vi "A170316-11-Main-large.vi"() -> ()   [LabVIEW 2020]
uses:
  System.Windows.Forms
  Global_Variable/Global.vi
  Database/Global1.vi
  <userlib>/_MGI/Menu Building/MenuTypes/MenuStrip/MGI_MenuStrip.lvclass
  <userlib>/_MGI/Menu Building/MenuItemStatusChange/MGI_MenuItemStatusChange.lvclass
  Libraries/S7/S7.lvlib
panel:
  out "PLC":bool
  out "产品型号":string
  in  "质量报警":bool
  in  "设备缺料":bool
  in  "设备故障":bool
  out "结果字":string
  out "前序状态字":string
  out "前序状态":bool
  in  "菜单":refnum<k24>(container)
  out "检测结果":bool
  in  "批次信息":string[][](table)
  out "提示信息":string
  out "错误":bool
  out "时间字符串":string
  out "日期字符串":string
  out "自动":bool
  out "userStatus":string caption="用户状态"
  out "userName":string caption="用户名"
  out "合格数量":u32
  out "生产数量":u32
  out "追溯码":string
  out "connectionMode":string caption="联机类型"
  in  "更换产品":refnum<vi>
  # "总成检验"
  # "工艺流程"
  # "检测结果："
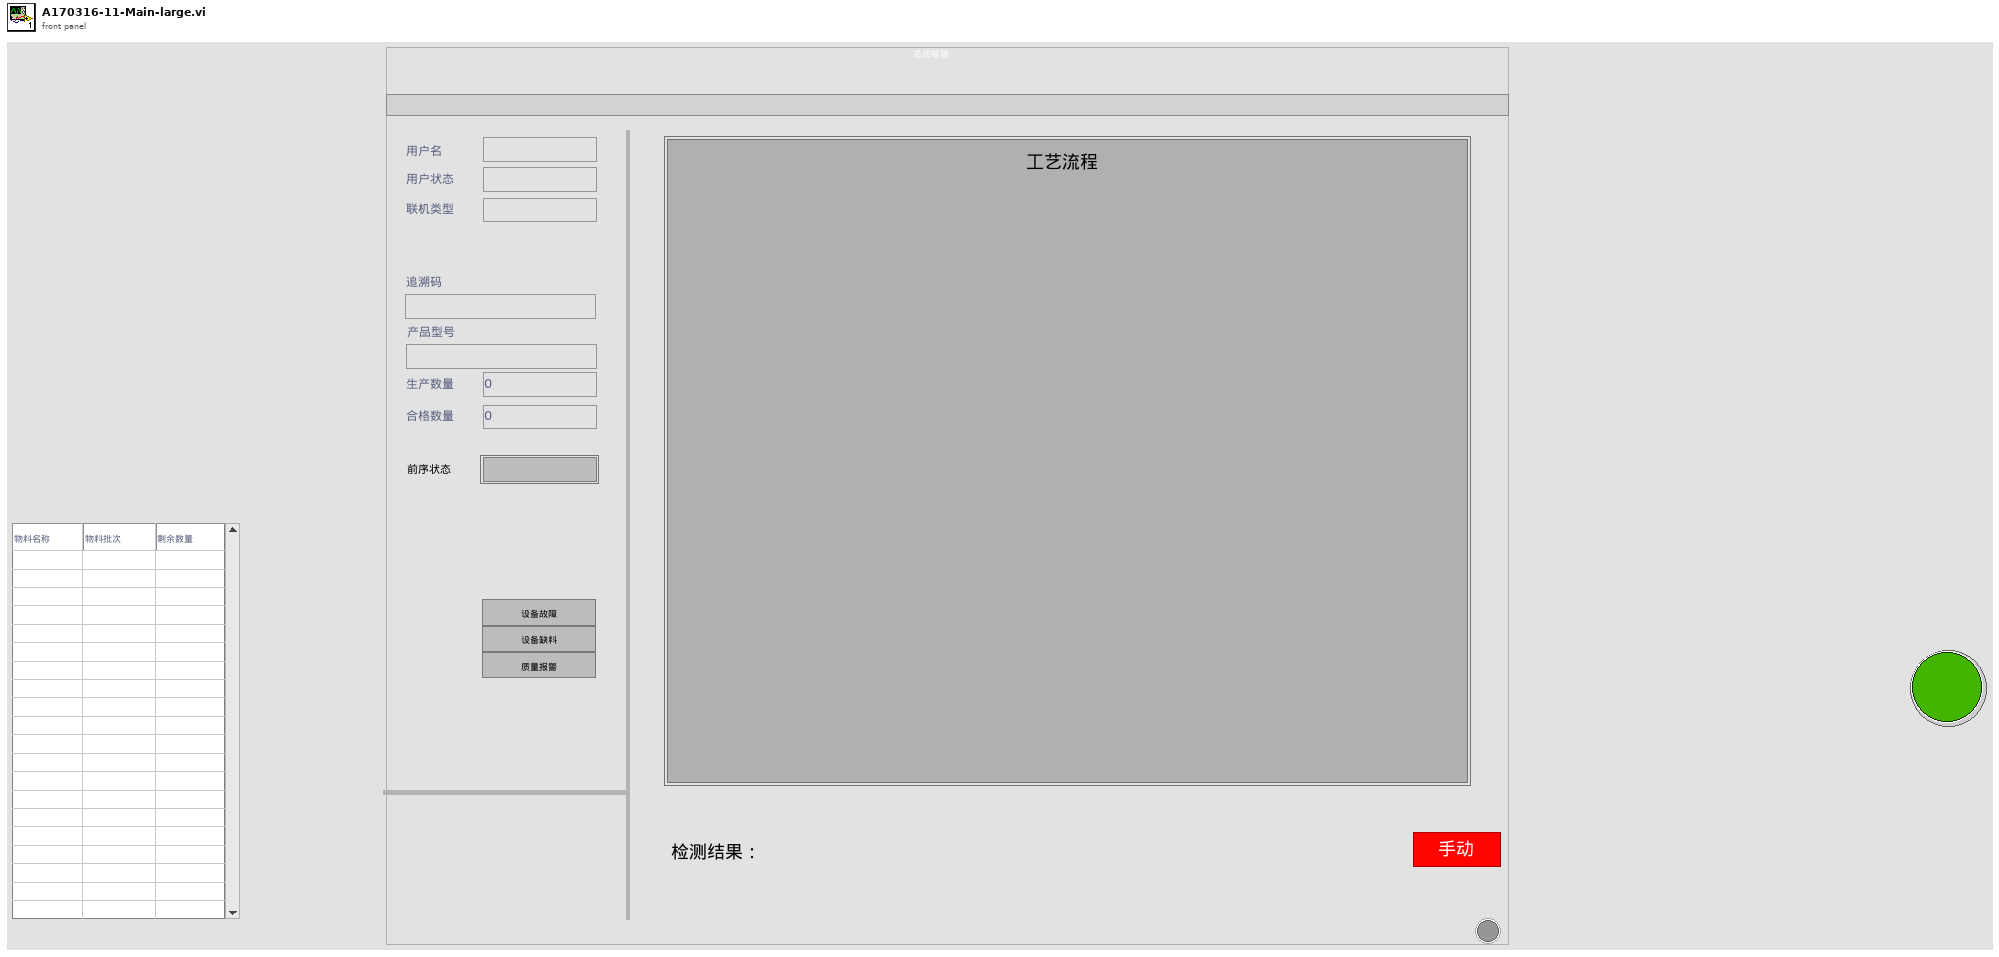
[diagram p1: front panel]
types:
  T1 = typedef "S7.lvlib/Broadcast Events--cluster.ctl" = cluster{"Module Did Init":refnum<user-event>, "Status Updated":refnum<user-event>, "Error Reported":refnum<user-event>, "Module Did Stop":refnum<user-event>, "Update Module Execution Status":refnum<user-event>}
  T2 = enum32{"Invalid", "Standard", "Closed", "Hidden", "Minimized", "Maximized"}
  T3 = enum32{"invalid app kind", "Development System", "Run Time System", "Student Edition", "Embedded LabVIEW", "Evaluation", "Custom"}
  T4 = cluster{"用户编号":string, "用户名":string, "用户密码(密文)":string, "用户权限":string}
  T5 = cluster{"Core":cluster{"Current VI Reference":refnum<vi>, "Close Panel on Exit?":bool}, "Your Boolean data":bool, "Your string data":string}
  T6 = cluster{"Current VI Reference":refnum<vi>, "Close Panel on Exit?":bool}
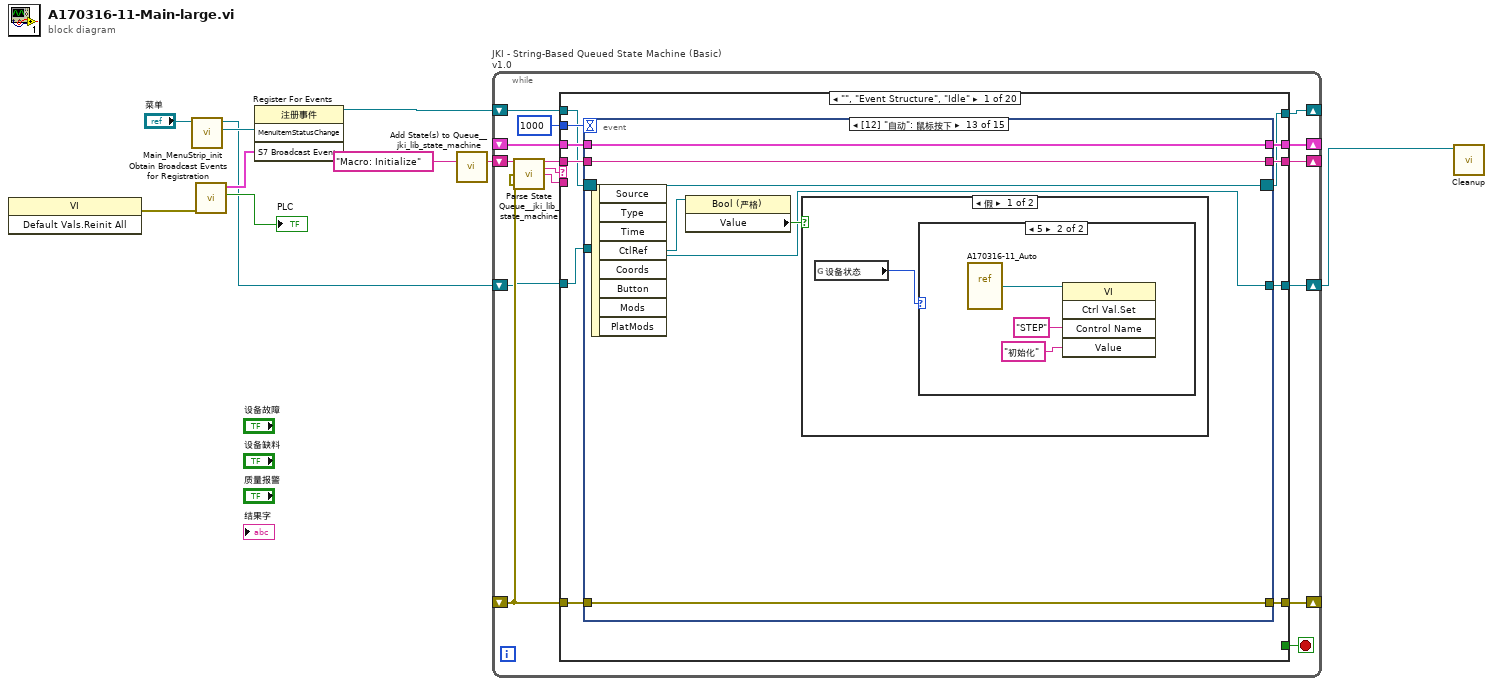
[diagram p0: block diagram]
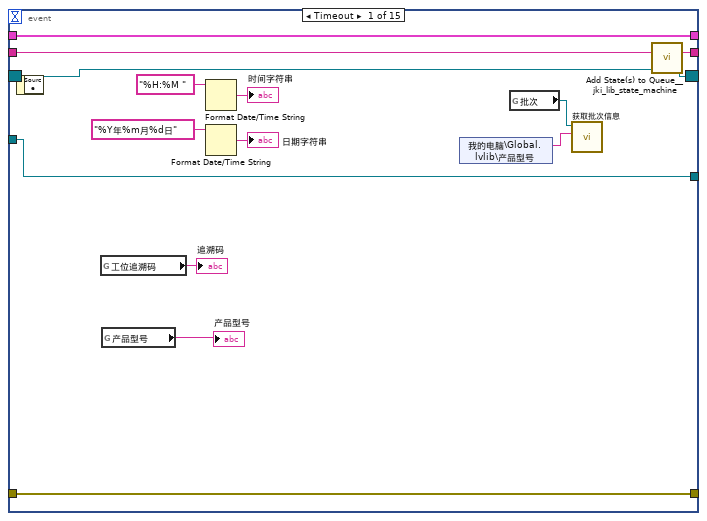
[diagram p2: hidden frame]
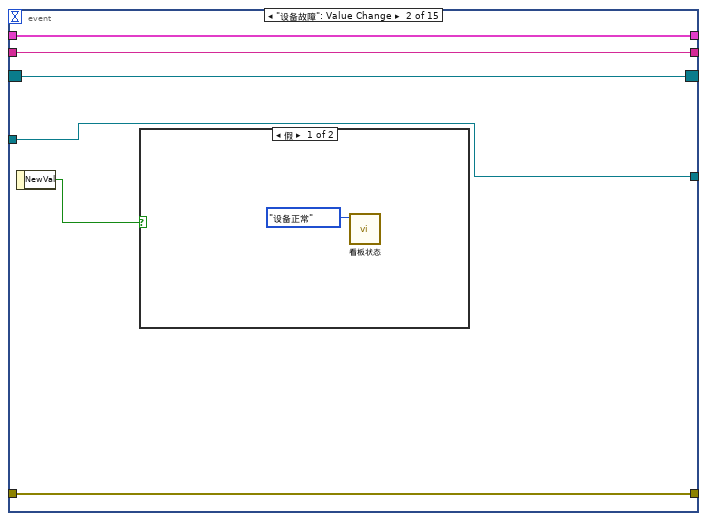
[diagram p3: hidden frame]
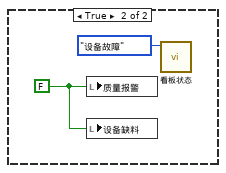
[diagram p4: hidden frame]
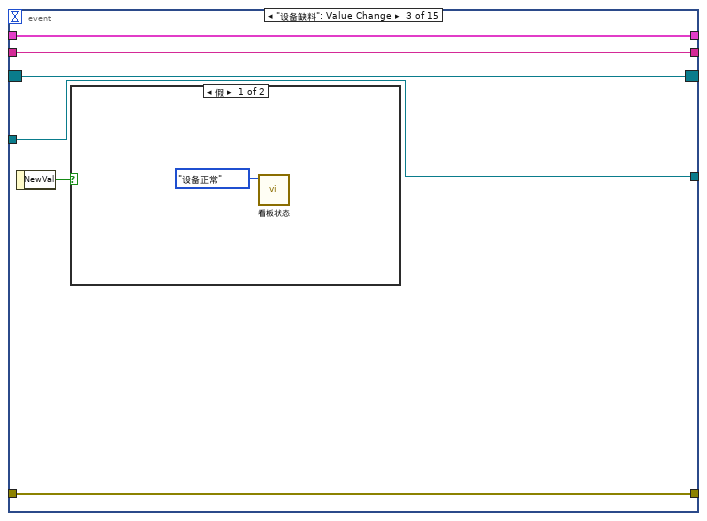
[diagram p5: hidden frame]
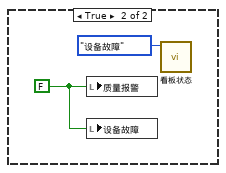
[diagram p6: hidden frame]
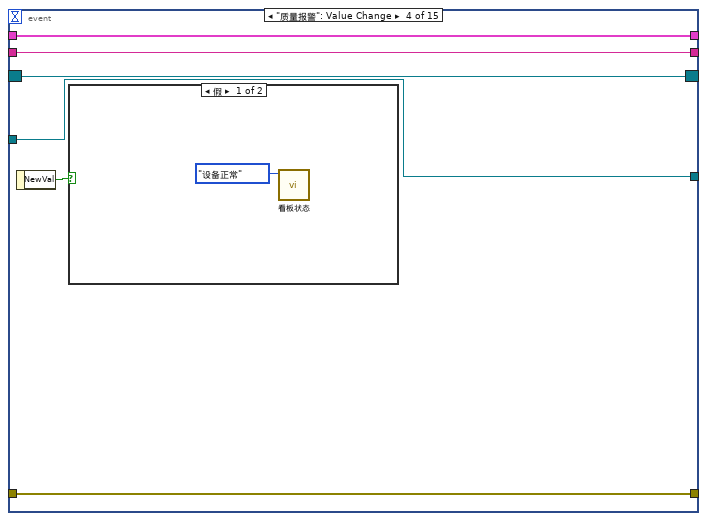
[diagram p7: hidden frame]
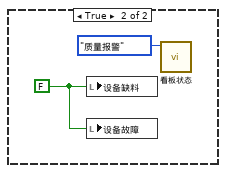
[diagram p8: hidden frame]
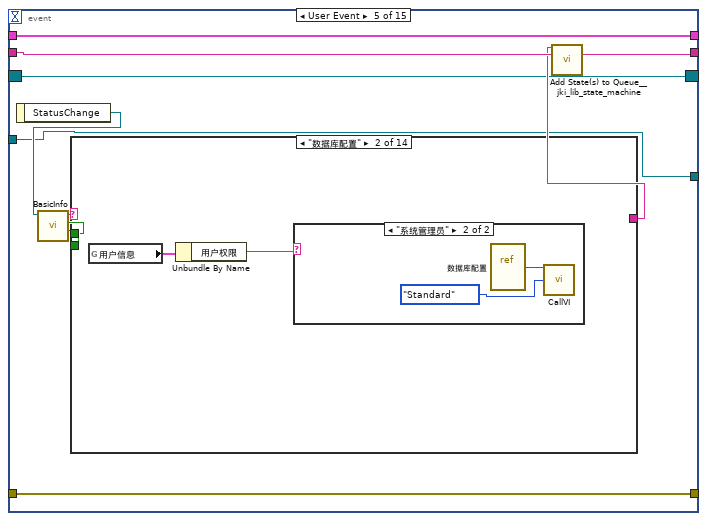
[diagram p9: hidden frame]
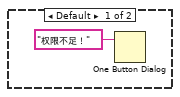
[diagram p11: hidden frame]
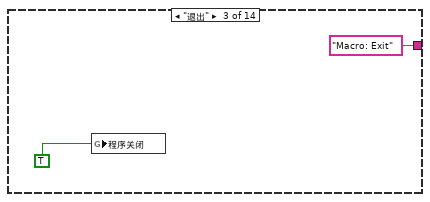
[diagram p12: hidden frame]
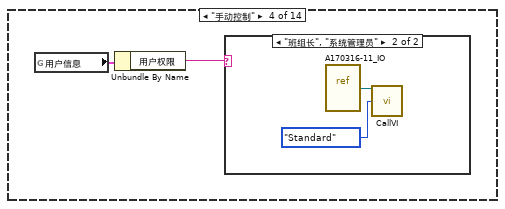
[diagram p13: hidden frame]
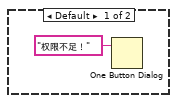
[diagram p14: hidden frame]
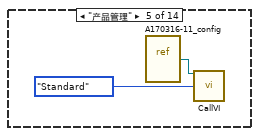
[diagram p15: hidden frame]
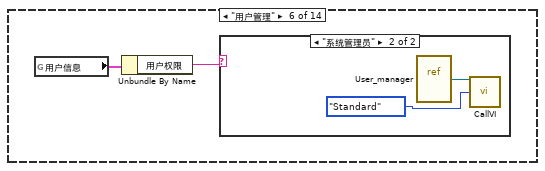
[diagram p16: hidden frame]
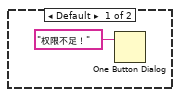
[diagram p17: hidden frame]
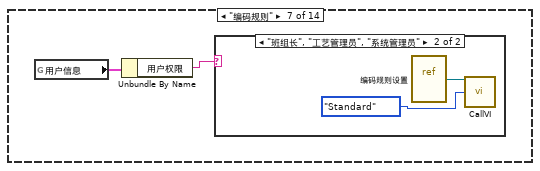
[diagram p18: hidden frame]
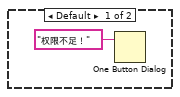
[diagram p19: hidden frame]
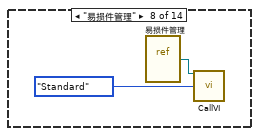
[diagram p20: hidden frame]
diagram:
  n1 = invoke class="VI" method="Default Vals.Reinit All"() -> (error out=w5:errorcluster)  [unwired: 3 in, 2 out]
  n2 = call "Main_MenuStrip_init.vi"("MenuStrip"="菜单") -> ("MenuItemStatusChange"=w7:refnum<user-event>, "Menu out"=w2:refnum<class "MGI_MenuStrip.lvclass">)  [unwired: 9 in]
  n3 = call "Obtain Broadcast Events for Registration.vi"("error in (no error)"=w5) -> ("Already running?"=→"PLC":bool, "S7 Broadcast Events"=w4:T1)  [unwired: 8 in, 1 out]
  n4 = register-events(w7, w4) -> (reference out=w6:refnum<event-registration>)  [unwired: 2 in, 1 out]
  n5 = call <vilib>:"Add State(s) to Queue__jki_lib_state_machine.vi"("State(s) in (\"\")"="Macro: Initialize") -> ("States Out"=w10:string)  [unwired: 14 in]
  n6 = while "JKI - String-Based Queued State Machine (Basic) v1.0" {
    shift-right: [w18] -> _
    shift-left: _ -> [w17]
    shift-right: [w21] -> _
    shift-left: _ -> [w15]
    shift-right: [w20] -> _
    shift-left: w10 -> [w22]
    shift-right: [w12] -> w1
    shift-left: w2 -> [w13]
    shift-right: [w11] -> _
    shift-left: w6 -> [w14]
    stop <- w19 stop-if-true
    n7 = call <vilib>:"Parse State Queue__jki_lib_state_machine.vi"("State Queue"=w22, "Error In (no error)"=w15) -> ("Remaining States"=w24:string, "Current State"=w25:string, "Arguments"=w23:string)  [unwired: 11 in]
    n8 = case shown="\"\", \"Event Structure\", \"Idle\"" w25 {
      selector: w25 -> [_ _ w281 _ _ _ _ _ _ _ _ _ _ _ _ _ _ _ _ _]
      tunnel: w24 -> [w36 w278 w285 w305 w313 w320 w326 w335 w343 w349 w363 w369 w415 w428 w456 w463 w477 w483 w489 w495]
      tunnel: w23 -> [_ _ _ _ _ _ _ _ _ _ _ _ w410 w422 _ _ _ _ _ _]
      tunnel: w17 -> [w34 w275 w283 w296 w310 w318 w323 _ w338 w346 w361 w367 w413 w424 w453 w460 w474 w480 w486 w492]
      tunnel: [w33 w276 w287 w302 errorcluster {"status"=FALSE, "code"=0, "source"=""} ("error out") w317 w324 w332 w339 w347 w358 w366 w411 w425 w454 w461 w475 w481 w487 w493] -> w21
      tunnel: w15 -> [w32 w276 w286 w302 w309 w317 w324 w332 w340 w347 w353 w366 w412 w426 w454 w461 w475 w481 w487 w493]
      tunnel: [w35 w277 w284 w304 w312 w319 w325 w334 w342 w348 w362 w368 w414 w427 w455 w462 w476 w482 w488 w494] -> w20
      tunnel: [_ _ _ _ _ TRUE _ _ _ _ _ _ _ _ _ _ _ _ _ _] -> w19
      tunnel: [w31 w275 w283 w303 w310 w318 w323 w333 w338 w346 w361 w367 w413 w424 w453 w460 w474 w480 w486 w492] -> w18
      tunnel: 1000 ("Timeout") -> [w30 _ _ _ _ _ _ _ _ _ _ _ _ _ _ _ _ _ _ _]
      tunnel: w14 -> [w29 w273 w280 w293 w307 w315 w322 w328 w337 w345 w351 w365 w409 w421 w452 w458 w464 w478 w485 w490]
      tunnel: w13 -> [w28 w274 w279 w292 w306 w314 w321 w327 w336 w344 w350 w364 w408 w420 w451 w457 w465 w479 w484 w491]
      tunnel: [w27 w274 w279 w292 w306 w314 w321 w327 w336 w344 w350 w364 w408 w420 w451 w457 w465 w479 w484 w491] -> w12
      tunnel: [w26 w273 w280 w293 w307 w315 w322 w328 w337 w345 w351 w365 w409 w421 w452 w458 w464 w478 w485 w490] -> w11
      frame "", "Event Structure", "Idle" {
        n9 = event shown="[12] \"自动\": 鼠标按下" {
          selector: w29 -> [w38 w51 w61 w70 w79 w147 w152 w159 w166 w175 w181 w232 w240 w257 w266]
          dyn-events: [w38 w51 w61 w70 w79 w145 w152 w159 w166 w175 w181 w232 w240 w257 w266] -> w26
          timeout: w30 -> [_ _ _ _ _ _ _ _ _ _ _ _ _ _ _]
          tunnel: w36 -> [w50 w54 w63 w72 w83 w137 w154 w161 w168 w177 w184 w236 w244 w264 w269]
          tunnel: [w49 w54 w63 w72 w82 w137 w153 w160 w167 w176 w182 w237 w244 w263 w270] -> w35
          tunnel: w34 -> [w47 w55 w64 w73 w84 w138 w155 w162 w169 w178 w183 w238 w245 w261 w272]
          tunnel: [w48 w53 w62 w71 w80 w139 w150 w157 w165 w171 w185 w235 w243 w262 w271] -> w33
          tunnel: w32 -> [w48 w53 w62 w71 w80 w149 w150 w157 w165 w172 w185 w235 w243 w262 w271]
          tunnel: [w47 w55 w64 w73 w84 w138 w155 w162 w169 w178 w183 w238 w245 w261 w272] -> w31
          tunnel: w28 -> [w37 w52 w60 w69 w78 w136 w156 w163 w170 w179 w180 w231 w239 w256 w265]
          tunnel: [w37 w52 w60 w69 w78 w136 w156 w163 w170 w179 w180 w231 w239 w256 w265] -> w27
          event Timeout {
            n10 = event-data() -> ()  [unwired: 1 in, 1 out]
            n11 = global read "Global1.vi" "工位追溯码"() -> (→"追溯码":string)
            n12 = global read "Global.vi" "产品型号"() -> (→"产品型号":string)
            n13 = Format Date/Time String(time format string (%c)="%H:%M ") -> (date/time string=→"时间字符串":string)  [unwired: 2 in]
            n14 = Format Date/Time String(time format string (%c)="%Y年%m月%d日") -> (date/time string=→"日期字符串":string)  [unwired: 2 in]
            n15 = shared-variable "我的电脑\\Global.lvlib\\产品型号"() -> (w42:string)  [unwired: 1 in, 1 out]
            n16 = global read "Global.vi" "批次"() -> (w41:refnum<vi>)
            n17 = call "获取批次信息.vi"("产品型号"=w42, "Tbl引用句柄"=w41) -> ()  [unwired: 8 in, 2 out]
            n18 = call <vilib>:"Add State(s) to Queue__jki_lib_state_machine.vi"("State(s) in (\"\")"=w50) -> ("States Out"=w49:string)  [unwired: 14 in]
          }
          event "设备故障": Value Change {
            n19 = event-data() -> ("NewVal"=w56:bool)  [unwired: 1 in]
            n20 = case shown="假" w56 {
              frame False {
                n21 = call "看板状态.vi"("设备状态"=enum16{"设备离线", "设备正常", "设备缺料", "设备故障", "质量报警"}."设备正常") -> ()  [unwired: 10 in, 1 out]
              }
              frame True {
                w58 = FALSE ("质量报警")
                n22 = local write "质量报警"(w58) -> ()
                n23 = local write "设备缺料"(w58) -> ()
                n24 = call "看板状态.vi"("设备状态"=enum16{"设备离线", "设备正常", "设备缺料", "设备故障", "质量报警"}."设备故障") -> ()  [unwired: 10 in, 1 out]
              }
            }
          }
          event "设备缺料": Value Change {
            n25 = event-data() -> ("NewVal"=w65:bool)  [unwired: 1 in]
            n26 = case shown="假" w65 {
              frame False {
                n27 = call "看板状态.vi"("设备状态"=enum16{"设备离线", "设备正常", "设备缺料", "设备故障", "质量报警"}."设备正常") -> ()  [unwired: 10 in, 1 out]
              }
              frame True {
                w67 = FALSE ("质量报警")
                n28 = local write "质量报警"(w67) -> ()
                n29 = local write "设备故障"(w67) -> ()
                n30 = call "看板状态.vi"("设备状态"=enum16{"设备离线", "设备正常", "设备缺料", "设备故障", "质量报警"}."设备故障") -> ()  [unwired: 10 in, 1 out]
              }
            }
          }
          event "质量报警": Value Change {
            n31 = event-data() -> ("NewVal"=w74:bool)  [unwired: 1 in]
            n32 = case shown="假" w74 {
              frame False {
                n33 = call "看板状态.vi"("设备状态"=enum16{"设备离线", "设备正常", "设备缺料", "设备故障", "质量报警"}."设备正常") -> ()  [unwired: 10 in, 1 out]
              }
              frame True {
                w76 = FALSE ("质量报警")
                n34 = local write "设备缺料"(w76) -> ()
                n35 = local write "设备故障"(w76) -> ()
                n36 = call "看板状态.vi"("设备状态"=enum16{"设备离线", "设备正常", "设备缺料", "设备故障", "质量报警"}."质量报警") -> ()  [unwired: 10 in, 1 out]
              }
            }
          }
          event User Event {
            n37 = event-data() -> ("StatusChange"=w85:refnum<class "MGI_MenuItemStatusChange.lvclass">)  [unwired: 1 in]
            n38 = call <userlib>:"BasicInfo.vi"("MGI_MenuItemStatusChange in"=w85) -> ("Enabled?"=w88:bool, "Checked?"=w87:bool, "Tag"=w86:string)  [unwired: 7 in, 1 out]
            n39 = case shown="\"数据库配置\"" w86 {
              tunnel: w87 -> [_ _ _ _ _ _ _ _ _ _ _ _ _ _]
              tunnel: w88 -> [_ _ _ _ _ _ _ _ _ _ _ _ _ _]
              tunnel: [_ _ "Macro: Exit" _ _ _ _ _ _ _ _ _ _ _] -> w81
              frame Default {
              }
              frame "数据库配置" {
                n40 = global read "Global1.vi" "用户信息"() -> (w89:T4)
                n41 = Unbundle By Name(w89) -> ("用户权限"=w90:string)
                n42 = case shown="\"系统管理员\"" w90 {
                  frame Default {
                    n43 = One Button Dialog(message="权限不足！" ("消息")) -> ()  [unwired: 1 in, 1 out]
                  }
                  frame "系统管理员" {
                    n44 = vi-ref "数据库配置.vi"() -> (w93:refnum<vi>)
                    n45 = call "CallVI.vi"("VI引用"=w93, "状态"=T2."Standard") -> ()  [unwired: 11 in, 3 out]
                  }
                }
              }
              frame "退出" {
                n46 = global write "Global.vi" "程序关闭"(TRUE ("程序关闭")) -> ()
              }
              frame "手动控制" {
                n47 = global read "Global1.vi" "用户信息"() -> (w97:T4)
                n48 = Unbundle By Name(w97) -> ("用户权限"=w96:string)
                n49 = case shown="\"班组长\", \"系统管理员\"" w96 {
                  frame Default {
                    n50 = One Button Dialog(message="权限不足！" ("消息")) -> ()  [unwired: 1 in, 1 out]
                  }
                  frame "班组长", "系统管理员" {
                    n51 = vi-ref "A170316-11_IO.vi"() -> (w100:refnum<vi>)
                    n52 = call "CallVI.vi"("VI引用"=w100, "状态"=T2."Standard") -> ()  [unwired: 11 in, 3 out]
                  }
                }
              }
              frame "产品管理" {
                n53 = vi-ref "A170316-11_config.vi"() -> (w102:refnum<vi>)
                n54 = call "CallVI.vi"("VI引用"=w102, "状态"=T2."Standard") -> ()  [unwired: 11 in, 3 out]
              }
              frame "用户管理" {
                n55 = global read "Global1.vi" "用户信息"() -> (w104:T4)
                n56 = Unbundle By Name(w104) -> ("用户权限"=w103:string)
                n57 = case shown="\"系统管理员\"" w103 {
                  frame Default {
                    n58 = One Button Dialog(message="权限不足！" ("消息")) -> ()  [unwired: 1 in, 1 out]
                  }
                  frame "系统管理员" {
                    n59 = vi-ref "User_manager.vi"() -> (w107:refnum<vi>)
                    n60 = call "CallVI.vi"("VI引用"=w107, "状态"=T2."Standard") -> ()  [unwired: 11 in, 3 out]
                  }
                }
              }
              frame "编码规则" {
                n61 = global read "Global1.vi" "用户信息"() -> (w109:T4)
                n62 = Unbundle By Name(w109) -> ("用户权限"=w108:string)
                n63 = case shown="\"班组长\", \"工艺管理员\", \"系统管理员\"" w108 {
                  frame Default {
                    n64 = One Button Dialog(message="权限不足！" ("消息")) -> ()  [unwired: 1 in, 1 out]
                  }
                  frame "班组长", "工艺管理员", "系统管理员" {
                    n65 = vi-ref "编码规则设置.vi"() -> (w112:refnum<vi>)
                    n66 = call "CallVI.vi"("VI引用"=w112, "状态"=T2."Standard") -> ()  [unwired: 11 in, 3 out]
                  }
                }
              }
              frame "易损件管理" {
                n67 = vi-ref "易损件管理.vi"() -> (w114:refnum<vi>)
                n68 = call "CallVI.vi"("VI引用"=w114, "状态"=T2."Standard") -> ()  [unwired: 11 in, 3 out]
              }
              frame "物料批次管理" {
                n69 = vi-ref "批次管理.vi"() -> (w116:refnum<vi>)
                n70 = call "CallVI.vi"("VI引用"=w116, "状态"=T2."Standard") -> ()  [unwired: 11 in, 3 out]
              }
              frame "报表" {
                n71 = call "文件对话框2"("start path"=path "D:/report", "prompt"="打开报表", "pattern (all files)"="*.doc;*.docx", "pattern label"="Word 文档") -> ("selected path"=w117:path, "error out"=w118:errorcluster)  [unwired: 8 in, 2 out]
                n72 = case shown="无错误" w118 {
                  selector: w118 -> [w124 w126]
                  tunnel: w117 -> [w125 _]
                  frame No Error {
                    w123 = 1 items=["Normal", "Maximize", "Minimize"] ("cpubbs_WindowState")
                    n73 = call "Open_Word.vi"("File Path"=w125, "cpubbs_WindowState"=w123, "错误输入（无错误）"=w124) -> ()  [unwired: 12 in, 1 out]
                  }
                  frame Error {
                    n74 = call <vilib>:"Clear Errors.vi"("error in (no error)"=w126) -> ()  [unwired: 5 in, 2 out]
                  }
                }
              }
              frame "报警信息" {
                n75 = vi-ref "报警信息.vi"() -> (w128:refnum<vi>)
                n76 = call "CallVI.vi"("VI引用"=w128, "状态"=T2."Standard") -> ()  [unwired: 11 in, 3 out]
              }
              frame "关于" {
                n77 = vi-ref "About.vi"() -> (w130:refnum<vi>)
                n78 = call "CallVI.vi"("VI引用"=w130, "状态"=T2."Standard") -> ()  [unwired: 11 in, 3 out]
              }
              frame "设备管理" {
                n79 = vi-ref "注册设备.vi"() -> (w132:refnum<vi>)
                n80 = call "CallVI.vi"("VI引用"=w132, "状态"=T2."Standard") -> ()  [unwired: 11 in, 3 out]
              }
              frame "操作演示" {
                n81 = call <vilib>:"Application Directory.vi"() -> ("Application Directory"=w135:path)
                n82 = Build Path(base path=w135, name or relative path="操作演示" ("名称或相对路径")) -> (appended path=w134:path)
                n83 = call "自动播放ppt.vi"("路径"=w134) -> ()  [unwired: 10 in, 1 out]
              }
            }
            n84 = call <vilib>:"Add State(s) to Queue__jki_lib_state_machine.vi"("State(s) in Front (\"\")"=w81, "State(s) in (\"\")"=w83) -> ("States Out"=w82:string)  [unwired: 13 in]
          }
          event "PLC": Value Change; "PLC": Mouse Down {
            n85 = event-data() -> ()  [unwired: 1 in, 4 out]
            n86 = call "Start Module.vi"("error in (no error)"=w149) -> ("Wait for Event Sync?"=w143:bool, "S7 Broadcast Events"=w146:T1, "Module Was Already Running?"=w148:bool)  [unwired: 7 in, 1 out]
            n87 = local write "PLC"(w148) -> ()
            n88 = register-events(reference=w147, w146) -> (reference out=w145:refnum<event-registration>, error out=w144:errorcluster)  [unwired: 2 in]
            n89 = call "Synchronize Module Events.vi"("error in (no error)"=w144, "Wait for Event Sync?"=w143) -> ("error out"=w142:errorcluster)  [unwired: 9 in]
            n90 = call "Init S7 Link.vi"("error in (no error)"=w142, "超时"=1000, "IP"="192.168.0.91") -> ("error out"=w139:errorcluster)  [unwired: 8 in]
          }
          event User Event {
            n91 = event-data() -> ("Init?"=w151:bool)  [unwired: 1 in, 1 out]
            n92 = local write "PLC"(w151) -> ()
            n93 = call <vilib>:"Add State(s) to Queue__jki_lib_state_machine.vi"("State(s) in (\"\")"=w154) -> ("States Out"=w153:string)  [unwired: 14 in]
          }
          event User Event {
            n94 = event-data() -> ("Running?"=w158:bool)  [unwired: 1 in]
            n95 = local write "PLC"(w158) -> ()
            n96 = call <vilib>:"Add State(s) to Queue__jki_lib_state_machine.vi"("State(s) in (\"\")"=w161) -> ("States Out"=w160:string)  [unwired: 14 in]
          }
          event User Event {
            n97 = event-data() -> ()  [unwired: 1 in, 3 out]
            n98 = local write "PLC"(FALSE ("PLC")) -> ()
            n99 = call <vilib>:"Add State(s) to Queue__jki_lib_state_machine.vi"("State(s) in (\"\")"=w168) -> ("States Out"=w167:string)  [unwired: 14 in]
          }
          event User Event {
            n100 = event-data() -> ("Error"=w173:errorcluster)  [unwired: 1 in, 2 out]
            n101 = Merge Errors(w173, w172) -> (w171:errorcluster)
            n102 = call <vilib>:"Add State(s) to Queue__jki_lib_state_machine.vi"("State(s) in Front (\"\")"="S7: Initialize\nIdle" ("State(s) in Front (\"\")"), "State(s) in (\"\")"=w177) -> ("States Out"=w176:string)  [unwired: 13 in]
          }
          event Menu Selection (User) {
            n103 = event-data() -> ("ItemTag"=w186:string)  [unwired: 1 in, 6 out]
            n104 = case shown="\"退出\"" w186 {
              frame "假", Default {
              }
              frame "数据库配置" {
                n105 = shared-variable "我的电脑\\Global.lvlib\\操作者权限"() -> (w187:string)  [unwired: 1 in, 1 out]
                n106 = case shown="\"系统管理员\"" w187 {
                  frame Default {
                    n107 = One Button Dialog(message="权限不足！" ("消息")) -> ()  [unwired: 1 in, 1 out]
                  }
                  frame "系统管理员" {
                    n108 = vi-ref "数据库配置.vi"() -> (w190:refnum<vi>)
                    n109 = call "CallVI.vi"("VI引用"=w190, "状态"=T2."Standard") -> ()  [unwired: 11 in, 3 out]
                  }
                }
              }
              frame "退出" {
                n110 = Quit LabVIEW() -> ()  [unwired: 1 in]
              }
              frame "手动控制" {
                n111 = shared-variable "我的电脑\\Global.lvlib\\操作者权限"() -> (w191:string)  [unwired: 1 in, 1 out]
                n112 = case shown="\"班组长\", \"系统管理员\"" w191 {
                  frame Default {
                    n113 = One Button Dialog(message="权限不足！" ("消息")) -> ()  [unwired: 1 in, 1 out]
                  }
                  frame "班组长", "系统管理员" {
                    n114 = vi-ref "A170316-11_IO.vi"() -> (w194:refnum<vi>)
                    n115 = call "CallVI.vi"("VI引用"=w194, "状态"=T2."Standard") -> ()  [unwired: 11 in, 3 out]
                  }
                }
              }
              frame "半自动控制" {
                n116 = disable-structure shown="禁用" {
                  frame Disabled {
                    n117 = shared-variable "我的电脑\\Global.lvlib\\操作者权限"() -> (w195:string)  [unwired: 1 in, 1 out]
                    n118 = case shown="\"班组长\", \"系统管理员\"" w195 {
                      frame Default {
                        n119 = One Button Dialog(message="权限不足！" ("消息")) -> ()  [unwired: 1 in, 1 out]
                      }
                      frame "班组长", "系统管理员" {
                        n120 = call "CallVI.vi"("VI引用"=refnum<vi> refnum, "状态"=T2."Maximized") -> ()  [unwired: 11 in, 3 out]
                      }
                    }
                  }
                  frame Enabled {
                    n121 = One Button Dialog(message="当前设备不具备半自动功能！" ("消息")) -> ()  [unwired: 1 in, 1 out]
                  }
                }
              }
              frame "产品管理" {
                n122 = vi-ref "A170316-11_config.vi"() -> (w201:refnum<vi>)
                n123 = call "CallVI.vi"("VI引用"=w201, "状态"=T2."Standard") -> ()  [unwired: 11 in, 3 out]
              }
              frame "系统配置" {
              }
              frame "用户管理" {
                n124 = shared-variable "我的电脑\\Global.lvlib\\操作者权限"() -> (w202:string)  [unwired: 1 in, 1 out]
                n125 = case shown="\"系统管理员\"" w202 {
                  frame Default {
                    n126 = One Button Dialog(message="权限不足！" ("消息")) -> ()  [unwired: 1 in, 1 out]
                  }
                  frame "系统管理员" {
                    n127 = vi-ref "User_manager.vi"() -> (w205:refnum<vi>)
                    n128 = call "CallVI.vi"("VI引用"=w205, "状态"=T2."Standard") -> ()  [unwired: 11 in, 3 out]
                  }
                }
              }
              frame "编码规则" {
                n129 = shared-variable "我的电脑\\Global.lvlib\\操作者权限"() -> (w206:string)  [unwired: 1 in, 1 out]
                n130 = case shown="\"班组长\", \"工艺管理员\", \"系统管理员\"" w206 {
                  frame Default {
                    n131 = One Button Dialog(message="权限不足！" ("消息")) -> ()  [unwired: 1 in, 1 out]
                  }
                  frame "班组长", "工艺管理员", "系统管理员" {
                    n132 = vi-ref "编码规则设置.vi"() -> (w209:refnum<vi>)
                    n133 = call "CallVI.vi"("VI引用"=w209, "状态"=T2."Standard") -> ()  [unwired: 11 in, 3 out]
                  }
                }
              }
              frame "易损件管理" {
                n134 = vi-ref "易损件管理.vi"() -> (w211:refnum<vi>)
                n135 = call "CallVI.vi"("VI引用"=w211, "状态"=T2."Standard") -> ()  [unwired: 11 in, 3 out]
              }
              frame "物料批次管理" {
                n136 = vi-ref "批次管理.vi"() -> (w213:refnum<vi>)
                n137 = call "CallVI.vi"("VI引用"=w213, "状态"=T2."Standard") -> ()  [unwired: 11 in, 3 out]
              }
              frame "打开报表" {
                n138 = call "文件对话框"("start path"=path "D:/report", "prompt"="打开报表", "pattern (all files)"="*.doc;*.docx", "pattern label"="Word 文档") -> ("selected path"=w214:path, "error out"=w215:errorcluster)  [unwired: 8 in, 2 out]
                n139 = case shown="无错误" w215 {
                  selector: w215 -> [w221 w223]
                  tunnel: w214 -> [w222 _]
                  frame No Error {
                    w220 = 1 items=["Normal", "Maximize", "Minimize"] ("cpubbs_WindowState")
                    n140 = call "Open_Word.vi"("File Path"=w222, "cpubbs_WindowState"=w220, "错误输入（无错误）"=w221) -> ()  [unwired: 12 in, 1 out]
                  }
                  frame Error {
                    n141 = call <vilib>:"Clear Errors.vi"("error in (no error)"=w223) -> ()  [unwired: 5 in, 2 out]
                  }
                }
              }
              frame "报警信息" {
                n142 = vi-ref "报警信息.vi"() -> (w225:refnum<vi>)
                n143 = call "CallVI.vi"("VI引用"=w225, "状态"=T2."Standard") -> ()  [unwired: 11 in, 3 out]
              }
              frame "关于" {
                n144 = vi-ref "About.vi"() -> (w227:refnum<vi>)
                n145 = call "CallVI.vi"("VI引用"=w227, "状态"=T2."Standard") -> ()  [unwired: 11 in, 3 out]
              }
              frame "操作演示" {
                n146 = call <vilib>:"Application Directory.vi"() -> ("Application Directory"=w230:path)
                n147 = Build Path(base path=w230, name or relative path="操作演示" ("名称或相对路径")) -> (appended path=w229:path)
                n148 = call "自动播放ppt.vi"("路径"=w229) -> ()  [unwired: 10 in, 1 out]
              }
            }
            n149 = call <vilib>:"Add State(s) to Queue__jki_lib_state_machine.vi"("State(s) in (\"\")"=w184) -> ("States Out"=w182:string)  [unwired: 14 in]
          }
          event "错误": Mouse Down {
            n150 = event-data() -> ()  [unwired: 1 in, 8 out]
            n151 = vi-ref "报警信息.vi"() -> (w234:refnum<vi>)
            n152 = call "CallVI.vi"("VI引用"=w234, "状态"=T2."Standard") -> ()  [unwired: 11 in, 3 out]
            n153 = call <vilib>:"Add State(s) to Queue__jki_lib_state_machine.vi"("State(s) in (\"\")"=w236) -> ("States Out"=w237:string)  [unwired: 14 in]
          }
          event "自动": Mouse Down {
            n154 = event-data() -> ("CtlRef"=w242:refnum<vi>)  [unwired: 1 in, 7 out]
            n155 = property class="Bool (严格)"(reference=w242) -> ("Value"=w241:bool)  [unwired: 1 in, 2 out]
            n156 = case shown="假" w241 {
              frame False {
                n157 = global read "Global.vi" "设备状态"() -> (w246:i32)
                n158 = case shown="5" w246 {
                  frame 0, Default {
                    n159 = call "浮动通知.vi"("通知内容"="请复位！") -> ()  [unwired: 11 in]
                  }
                  frame 5 {
                    n160 = vi-ref "A170316-11_Auto.vi"() -> (w250:refnum<vi>)
                    n161 = invoke class="VI" method="Ctrl Val.Set"(reference=w250, "Control Name"="STEP" ("控件名"), "Value"="初始化" ("控件名")) -> ()  [unwired: 2 in, 5 out]
                  }
                }
              }
              frame True {
                n162 = Two Button Dialog(message="自动程序运行中，\n是否切换为手动？" ("消息")) -> (T button?=w251:bool)  [unwired: 2 in]
                n163 = case shown="真" w251 {
                  frame False {
                  }
                  frame True {
                    n164 = vi-ref "A170316-11_Auto.vi"() -> (w255:refnum<vi>)
                    n165 = invoke class="VI" method="Ctrl Val.Set"(reference=w255, "Control Name"="STEP" ("控件名"), "Value"="手动" ("控件名")) -> ()  [unwired: 2 in, 5 out]
                  }
                }
              }
            }
          }
          event Panel Close? {
            n166 = event-data() -> ()  [unwired: 1 in, 1 out]
            n167 = global write "Global.vi" "程序关闭"(TRUE ("程序关闭")) -> ()
            n168 = event-data("Discard?"=TRUE) -> ()  [unwired: 1 in, 1 out]
            n169 = call <vilib>:"Add State(s) to Queue__jki_lib_state_machine.vi"("State(s) in Front (\"\")"="Macro: Exit", "State(s) in (\"\")"=w264) -> ("States Out"=w263:string)  [unwired: 13 in]
          }
          event "更换产品": Value Change {
            n170 = event-data() -> ("NewVal"=w268:refnum<vi>)  [unwired: 1 in, 5 out]
            n171 = control-ref of="子面板"() -> (w267:refnum<vi>)
            n172 = call "Call_SubPanal.vi"("VI引用句柄"=w268, "SubPnl引用句柄"=w267) -> ()  [unwired: 9 in, 1 out]
            n173 = call <vilib>:"Add State(s) to Queue__jki_lib_state_machine.vi"("State(s) in (\"\")"=w269) -> ("States Out"=w270:string)  [unwired: 14 in]
          }
        }
      }
      frame "---------- Core ----------" {
        n174 = call <vilib>:"Add State(s) to Queue__jki_lib_state_machine.vi"("State(s) in (\"\")"=w278) -> ("States Out"=w277:string)  [unwired: 14 in]
      }
      frame Default {
        w290 = 42 items=["No error", "Argument error", "Memory is full", "Out of zone", "End of file", "File already open", "Generic file I/O error", "File not found", "File permission error", "Disk is full", "Duplicate path", "Too many files open", "System feature not enabled", "Resource file not found", "Cannot add resource", "Resource not found", "Image not found", "Image memory error", "Pen does not exist", "Config type invalid", "Config token not found", "Config parse error", "Config memory error", "Bad external code format", "Bad external code offset", "External code not present", "Null window", "Destroy window error", "Null menu", "Print aborted", "Bad print record", "Print driver error", "Windows error during printing", "Memory error during printing", "Print dialog error", "Generic print error", "Invalid device refnum", "Device not found", "Device parameter error", "Device unit error", "Cannot open device", "Device call aborted", "Generic error", "Cancelled by user", "Object ID too low", "Object ID too high", "Object not in heap", "Unknown heap", "Unknown object (invalid DefProc)", "Unknown object (DefProc not in table)", "Message out of range", "Invalid (null) method", "Unknown message", "Manager call not supported", "Bad address", "Network operation in progress", "Network operation timed out", "Connection is busy", "Network attribute not supported", "Network error", "Address in use", "System out of memory", "Connection aborted", "Connection refused", "Not connected", "Already connected", "Connection closed", "Initialization error (interapplication manager)", "Bad occurrence", "Wait on unbound occurrence handler", "Occurrence queue overflow", "Datalog type conflict", "Unused", "Unrecognized type (interapplication manager)", "Memory corrupt", "Failed to make temporary DLL", "Old CIN version", "Drag socket not found", "Failed to load drop-object", "Failed to register OLE object", "Failed to release OLE object", "Format specifier type mismatch", "Unknown format specifier", "Too few format specifiers", "Too many format specifiers", "Scan failed", "Newer CIN version", "Error converting to variant", "Runtime menu error", "Password tampered", "Variant attribute not found", "Incompatible variant data type", "Event data is not available", "Event Store is not present", "Occurrence is not found", "Event Queue is not created", "Event info is not available", "Refnum passed is NULL", "Error retrieving Class GUID", "Error retrieving CoClass GUID", "Error retrieving TypeLib GUID.", "Bad built application magic bytes.", "Specific driver is different from the specific driver associated with the Logical Name.", "There is no session opened to the class driver.", "Max Error", "MAX - Error with config objects", "MAX - Error loading configuration", "MAX - Group not supported"]
        # "Current State"
        n175 = Format Into String(format string="Software Exception: Unhandled State \"%s\"." ("message"), error in=w286, w281) -> (resulting string=w289:string, error out=w288:errorcluster)  [unwired: 1 in]
        n176 = call <vilib>:"Error Cluster From Error Code.vi"("show call chain? (False)"=TRUE, "error in (no error)"=w288, "error message (\"\")"=w289, "error code (0)"=w290) -> ("error out"=w287:errorcluster)  [unwired: 5 in]
        n177 = call <vilib>:"Add State(s) to Queue__jki_lib_state_machine.vi"("State(s) in (\"\")"=w285) -> ("States Out"=w284:string)  [unwired: 14 in]
      }
      frame "Initialize Core Data" {
        # "originally closed?"
        # "exe?"
        n178 = property class="VI"() -> ("Front Panel.Open"=w301:bool)  [unwired: 2 in, 2 out]
        n179 = property class="App"() -> ("App.Kind"=w300:T3)  [unwired: 2 in, 2 out]
        n180 = control-ref of="Current VI Reference"() -> (w294:refnum<vi>)
        n181 = Not(x=w301) -> (.not. x?=w298:bool)
        n182 = Equal?(x=w300, y=T3."Run Time System" ("Application:Kind")) -> (x = y?=w297:bool)
        n183 = Or(x=w298, y=w297) -> (x .or. y?=w295:bool)
        n184 = Bundle By Name(cluster=w296, "Core.Current VI Reference"=w294, "Core.Close Panel on Exit?"=w295) -> (w303:T5)
        n185 = call <vilib>:"Add State(s) to Queue__jki_lib_state_machine.vi"("State(s) in (\"\")"=w305) -> ("States Out"=w304:string)  [unwired: 14 in]
      }
      frame "Error Handler" {
        n186 = call <vilib>:"General Error Handler.vi"("error in (no error)"=w309) -> ()  [unwired: 10 in, 5 out]
        n187 = call <vilib>:"Add State(s) to Queue__jki_lib_state_machine.vi"("State(s) in Front (\"\")"="/* Post Error States", "State(s) in (\"\")"=w313) -> ("States Out"=w312:string)  [unwired: 13 in]
      }
      frame "Exit" {
        n188 = call <vilib>:"Add State(s) to Queue__jki_lib_state_machine.vi"("State(s) in (\"\")"=w320) -> ("States Out"=w319:string)  [unwired: 14 in]
      }
      frame "---------- Data ----------" {
        n189 = call <vilib>:"Add State(s) to Queue__jki_lib_state_machine.vi"("State(s) in (\"\")"=w326) -> ("States Out"=w325:string)  [unwired: 14 in]
      }
      frame "Data: Initialize" {
        w329 = T6 {"Current VI Reference"=refnum, "Close Panel on Exit?"=FALSE}  # Core
        w331 = TRUE  # Your Boolean data
        w330 = ""  # Your string data
        n190 = Bundle("Core"=w329, "Your Boolean data"=w331, "Your string data"=w330) -> (w333:T5)  [unwired: 1 in]
        n191 = call <vilib>:"Add State(s) to Queue__jki_lib_state_machine.vi"("State(s) in (\"\")"=w335) -> ("States Out"=w334:string)  [unwired: 14 in]
      }
      frame "Data: Cleanup" {
        n192 = Unbundle By Name(w338) -> ("Core.Current VI Reference"=w341:refnum<vi>)
        n193 = Close Reference(reference=w341, error in (no error)=w340) -> (error out=w339:errorcluster)
        n194 = call <vilib>:"Add State(s) to Queue__jki_lib_state_machine.vi"("State(s) in (\"\")"=w343) -> ("States Out"=w342:string)  [unwired: 14 in]
      }
      frame "---------- UI ----------" {
        # "Do not put any code in this frame.\n(It is a separator no-op. You can make a copy of this frame to create a new UI frame)"
        n195 = call <vilib>:"Add State(s) to Queue__jki_lib_state_machine.vi"("State(s) in (\"\")"=w349) -> ("States Out"=w348:string)  [unwired: 14 in]
      }
      frame "UI: Initialize" {
        n196 = vi-ref "A170316-11_Auto.vi"() -> (w352:refnum<vi>)
        n197 = invoke on="子面板" class="SubPnl" method="Insert VI"(error in=w353, "VI Ref"=w352) -> (error out=w354:errorcluster)  [unwired: 2 in, 3 out]
        n198 = invoke class="VI" method="Run VI"(reference=w352, error in=w354, "Wait until done"=FALSE ("结束前等待"), "Auto Dispose Ref"=TRUE ("自动销毁引用")) -> (error out=w357:errorcluster)  [unwired: 1 in, 4 out]
        n199 = call "窗口自动调整.vi"("error in (no error)"=w357, "max？"=TRUE, "border spacing (2 px)"=0) -> ("error out"=w358:errorcluster)  [unwired: 3 in, 1 out]
        n200 = call <vilib>:"Add State(s) to Queue__jki_lib_state_machine.vi"("State(s) in (\"\")"=w363) -> ("States Out"=w362:string)  [unwired: 14 in]
      }
      frame "UI: Init" {
        n201 = stacked-sequence {
          frame #0 {
            w371 = FALSE ("已启用")
            n202 = Current VI's Menubar() -> (w373:refnum<k9>)
            n203 = Set Menu Item Info(7:"半自动控制" ("项标识符"), 9:w371, 11:w373) -> (0:w374:errorcluster, 3:w375:refnum<k9>)  [unwired: 4 in]
            n204 = Set Menu Item Info(7:"易损件管理" ("项标识符"), 8:w374, 9:w371, 11:w375) -> ()  [unwired: 3 in, 2 out]
          }
          frame #1 {
            w379 = u32 0 ("合格数量")
            (unwired) "" ("productsName")
            n205 = global read "Global1.vi" "联机模式"() -> (w376:enum16{"单机", "联网"})
            n206 = global write "Global1.vi" "工位追溯码"("" ("输出轴码")) -> ()
            n207 = case shown="\"联网\"" w376 {
              tunnel: ["联网" ("connectionMode") "单机" ("connectionMode")] -> w380
              frame "联网" {
              }
              frame "单机", Default {
              }
            }
            "connectionMode" <- w380
            "生产数量" <- w379
            "合格数量" <- w379
            "检测结果" <- FALSE ("检测结果")
          }
          frame #2 {
            n208 = control-ref of="合格数量"() -> (w387:refnum<vi>)
            n209 = control-ref of="批次信息"() -> (w393:refnum<vi>)
            n210 = control-ref of="生产数量"() -> (w388:refnum<vi>)
            n211 = control-ref of="前序状态字"() -> (w384:refnum<vi>)
            n212 = control-ref of="前序状态"() -> (w385:refnum<vi>)
            n213 = control-ref of="自动"() -> (w391:refnum<vi>)
            n214 = control-ref of="错误"() -> (w392:refnum<vi>)
            n215 = global write "Global.vi" "生产数量"(w388) -> ()
            n216 = global write "Global.vi" "合格数量"(w387) -> ()
            n217 = global write "Global.vi" "批次"(w393) -> ()
            n218 = global write "Global.vi" "报警图标"(w392) -> ()
            n219 = global write "Global.vi" "程序自动"(w391) -> ()
            n220 = global write "Global.vi" "前序状态显示字"(w384) -> ()
            n221 = global write "Global.vi" "前序状态"(w385) -> ()
            n222 = control-ref of="提示信息"() -> (w390:refnum<vi>)
            n223 = global write "Global.vi" "提示信息"(w390) -> ()
            n224 = control-ref of="结果字"() -> (w383:refnum<vi>)
            n225 = control-ref of="更换产品"() -> (w389:refnum<vi>)
            n226 = control-ref of="检测结果"() -> (w386:refnum<vi>)
            n227 = global write "Global.vi" "检测结果"(w386) -> ()
            n228 = global write "Global.vi" "结果显示字"(w383) -> ()
            n229 = global write "Global.vi" "更换产品"(w389) -> ()
          }
          frame #3 {
            n230 = global read "Global.vi" "前序状态显示字"() -> (w404:refnum<vi>)
            n231 = global read "Global.vi" "结果显示字"() -> (w400:refnum<vi>)
            n232 = vi-ref "A170316-11_config.vi"() -> (w406:refnum<vi>)
            n233 = call "CallVI.vi"("VI引用"=w406, "状态"=T2."Standard") -> ()  [unwired: 11 in, 3 out]
            n234 = property class="Str"(reference=w404, "Value"="" ("值")) -> ()  [unwired: 1 in, 2 out]
            n235 = property class="Str"(reference=w400, "Value"="..." ("值")) -> ()  [unwired: 1 in, 2 out]
            n236 = global read "Global.vi" "前序状态"() -> (w402:refnum<vi>)
            n237 = call "看板状态.vi"("附加信息"="", "设备状态"=enum16{"设备离线", "设备正常", "设备缺料", "设备故障", "质量报警"}."设备正常") -> ("错误输出"=w396:errorcluster)  [unwired: 9 in]
            n238 = vi-ref "client.vi"() -> (w397:refnum<vi>)
            n239 = call "Colour.vi"("result"="", "colourRef"=w402) -> ()  [unwired: 9 in, 1 out]
            n240 = call "浮动通知.vi"("通知内容"="请选择产品") -> ()  [unwired: 11 in]
            n241 = call "CallVI.vi"("VI引用"=w397, "状态"=T2."Hidden", "错误输入"=w396) -> ()  [unwired: 10 in, 3 out]
          }
        }
        n242 = call <vilib>:"Add State(s) to Queue__jki_lib_state_machine.vi"("State(s) in (\"\")"=w369) -> ("States Out"=w368:string)  [unwired: 14 in]
      }
      frame "UI: Cursor Set" {
        # "Argument"
        n243 = case shown="\"Idle\", 默认" w410 {
          tunnel: w412 -> [w417 w419]
          tunnel: [w416 w418] -> w411
          frame "Idle", Default {
            n244 = call <vilib>:"Unset Busy.vi"("error in (no error)"=w417) -> ("error out"=w416:errorcluster)  [unwired: 10 in]
          }
          frame "Busy" {
            n245 = call <vilib>:"Set Busy.vi"("error in (no error)"=w419) -> ("error out"=w418:errorcluster)  [unwired: 9 in, 1 out]
          }
        }
        n246 = call <vilib>:"Add State(s) to Queue__jki_lib_state_machine.vi"("State(s) in (\"\")"=w415) -> ("States Out"=w414:string)  [unwired: 14 in]
      }
      frame "UI: Front Panel State" {
        # "Argument"
        n247 = Unbundle By Name(w424) -> ("Core.Current VI Reference"=w423:refnum<vi>)
        n248 = case shown="\"Open\", 默认" w422 {
          tunnel: w426 -> [w432 w445]
          tunnel: [w434 w446] -> w425
          tunnel: w423 -> [w433 w443]
          frame "Open", Default {
            n249 = property class="VI"(reference=w433, error in=w432) -> (reference out=w430:refnum<vi>, error out=w431:errorcluster, "Front Panel.Open"=w429:bool)
            n250 = case shown="真" w429 {
              tunnel: [w437 w440] -> w434
              tunnel: w431 -> [w436 w440]
              tunnel: w430 -> [w435 _]
              frame False {
                n251 = invoke class="VI" method="FP.Open"(reference=w435, error in=w436, "Activate"=TRUE, "State"=T2."Standard") -> (error out=w437:errorcluster)  [unwired: 1 in, 4 out]
              }
              frame True {
              }
            }
          }
          frame "Close" {
            n252 = property class="VI"(reference=w443, error in=w445) -> (reference out=w442:refnum<vi>, error out=w444:errorcluster, "Front Panel.Open"=w441:bool)
            n253 = case shown="真" w441 {
              tunnel: [w447 w450] -> w446
              tunnel: w444 -> [w447 w449]
              tunnel: w442 -> [_ w448]
              frame False {
              }
              frame True {
                n254 = invoke class="VI" method="FP.Close"(reference=w448, error in=w449) -> (error out=w450:errorcluster)  [unwired: 1 in, 2 out]
              }
            }
          }
        }
        n255 = call <vilib>:"Add State(s) to Queue__jki_lib_state_machine.vi"("State(s) in (\"\")"=w428) -> ("States Out"=w427:string)  [unwired: 14 in]
      }
      frame "---------- Macro ----------" {
        n256 = call <vilib>:"Add State(s) to Queue__jki_lib_state_machine.vi"("State(s) in (\"\")"=w456) -> ("States Out"=w455:string)  [unwired: 14 in]
      }
      frame "Macro: Initialize" {
        w459 = "Data: Initialize\nInitialize Core Data\nUI: Initialize\nUI: Init\nUI: Front Panel State >> Open"  # Data: Initialize Initialize Core Data UI: Initialize UI: Init UI: Front Panel State >> Open
        n257 = call <vilib>:"Add State(s) to Queue__jki_lib_state_machine.vi"("State(s) in Front (\"\")"=w459, "State(s) in (\"\")"=w463) -> ("States Out"=w462:string)  [unwired: 13 in]
      }
      frame "Macro: Exit" {
        n258 = Unbundle By Name(w474) -> ("Core.Close Panel on Exit?"=w473:bool)
        n259 = vi-ref "client.vi"() -> (w467:refnum<vi>)
        n260 = invoke class="VI" method="FP.Close"(reference=w467) -> (reference out=w466:refnum<vi>)  [unwired: 2 in, 2 out]
        n261 = Close Reference(reference=w466) -> ()  [unwired: 1 in, 1 out]
        n262 = Select(t="UI: Front Panel State >> Close", s=w473, f="") -> (s? t:f=w470:string)
        n263 = call <vilib>:"Add State(s) to Queue__jki_lib_state_machine.vi"("State(s) in (\"\")"=w470, "State(s) at Back (\"\")"="Data: Cleanup\nExit") -> ("States Out"=w468:string)  [unwired: 13 in]
        n264 = call <vilib>:"Add State(s) to Queue__jki_lib_state_machine.vi"("State(s) in Front (\"\")"=w468, "State(s) in (\"\")"=w477) -> ("States Out"=w476:string)  [unwired: 13 in]
      }
      frame "---------- New Category ----------" {
        n265 = call <vilib>:"Add State(s) to Queue__jki_lib_state_machine.vi"("State(s) in (\"\")"=w483) -> ("States Out"=w482:string)  [unwired: 14 in]
      }
      frame "New Category: 1" {
        n266 = call <vilib>:"Add State(s) to Queue__jki_lib_state_machine.vi"("State(s) in (\"\")"=w489) -> ("States Out"=w488:string)  [unwired: 14 in]
      }
      frame "New Category: 2" {
        n267 = call <vilib>:"Add State(s) to Queue__jki_lib_state_machine.vi"("State(s) in (\"\")"=w495) -> ("States Out"=w494:string)  [unwired: 14 in]
      }
    }
  }
  n268 = call-dynamic "Cleanup.vi"("MenuStrip in"=w1) -> ()  [unwired: 10 in, 1 out]
